vi "Dresden R2R Sputter 03.02.2018 IY24.vi"() -> ()   [LabVIEW 2009] (continued)
                                frame #0 {
                                n24699 = local write "Pc_bv1_auto_open"(TRUE ("Pc_bv1_auto_open")) -> ()
                                }
                                frame #1 {
                                }
                                }
                                }
                                frame #1 {
                                }
                                }
                                }
                                frame #4 {
                                n24700 = local read "Semi"() -> (w30074:bool)
                                n24701 = case shown="False" w30074 {
                                frame #0 {
                                n24702 = local read "Pc_bv_opened_ch1"() -> (w30075:bool)
                                n24703 = case shown="False" w30075 {
                                frame #0 {
                                n24704 = Wait (ms)(milliseconds to wait=u32 1000) -> ()  [unwired: 1 out]
                                }
                                frame #1 {
                                }
                                }
                                }
                                frame #1 {
                                }
                                }
                                }
                                frame #5 {
                                n24705 = local read "Semi"() -> (w30077:bool)
                                n24706 = case shown="False" w30077 {
                                frame #0 {
                                n24707 = while {
                                i -> [w30083]
                                stop <- w30079 stop-if-true
                                n24708 = local read "Pc_bv_opened_ch1"() -> (w30081:bool)
                                n24709 = Greater?(x=w30083, y=120) -> (0:w30082:bool)
                                n24710 = local read "Semi"() -> (w30080:bool)
                                n24711 = Compound Arithmetic op=OR(w30080, w30081, w30082) -> (w30079:bool)
                                n24712 = Wait (ms)(milliseconds to wait=u32 500) -> ()  [unwired: 1 out]
                                }
                                }
                                frame #1 {
                                }
                                }
                                }
                                frame #6 {
                                n24713 = local read "Semi"() -> (w30085:bool)
                                n24714 = case shown="False" w30085 {
                                frame #0 {
                                n24715 = local read "Pc_bv_opened_ch1"() -> (w30086:bool)
                                n24716 = case shown="False" w30086 {
                                frame #0 {
                                n24717 = local write "Error Message"("Start up process  cancelled\nbecause  PC-BV not opened.\nPlease check PC-BV1 connections." ("Error Message")) -> ()
                                n24718 = Wait (ms)(milliseconds to wait=u32 1000) -> ()  [unwired: 1 out]
                                }
                                frame #1 {
                                }
                                }
                                }
                                frame #1 {
                                }
                                }
                                }
                                }
                                }
                                frame #1 {
                                }
                                }
                                }
                                frame #1 {
                                n24719 = local read "Semi"() -> (w30089:bool)
                                n24720 = case shown="False" w30089 {
                                frame #0 {
                                n24721 = Wait (ms)(milliseconds to wait=u32 1000) -> ()  [unwired: 1 out]
                                n24722 = local write "SMW19"(TRUE ("CMW16")) -> ()
                                }
                                frame #1 {
                                }
                                }
                                }
                                }
                                }
                                frame #16 {
                                # "set ar zero"
                                n24723 = stacked-sequence {
                                frame #0 {
                                n24724 = local read "Semi"() -> (w30092:bool)
                                n24725 = case shown="False" w30092 {
                                frame #0 {
                                n24726 = stacked-sequence {
                                frame #0 {
                                n24727 = local read "Semi"() -> (w30093:bool)
                                n24728 = case shown="False" w30093 {
                                frame #0 {
                                n24729 = local write "Ar_auto_set_zero_ch1"(TRUE ("Ar_auto_set_zero_ch1")) -> ()
                                }
                                frame #1 {
                                }
                                }
                                }
                                frame #1 {
                                n24730 = local read "Semi"() -> (w30095:bool)
                                n24731 = case shown="False" w30095 {
                                frame #0 {
                                n24732 = while {
                                i -> [w30098]
                                stop <- w30097 stop-if-true
                                n24733 = Greater?(x=w30098, y=150) -> (0:w30097:bool)
                                n24734 = local read "Semi"() -> (w30096:bool)
                                n24735 = case shown="False" w30096 {
                                tunnel: [FALSE TRUE] -> _
                                frame #0 {
                                n24736 = Wait Until Next ms Multiple(millisecond multiple=u32 200) -> ()  [unwired: 1 out]
                                }
                                frame #1 {
                                }
                                }
                                }
                                }
                                frame #1 {
                                }
                                }
                                }
                                frame #2 {
                                n24737 = local read "Semi"() -> (w30103:bool)
                                n24738 = case shown="False" w30103 {
                                frame #0 {
                                n24739 = local read "Ar_sccm_act 5"() -> (w30105:dbl)
                                n24740 = Less?(x=w30105, y=1) -> (x < y?=w30104:bool)
                                n24741 = case shown="False" w30104 {
                                frame #0 {
                                n24742 = local write "Ar_auto_set_zero_ch1"(TRUE ("Ar_auto_set_zero_ch1")) -> ()
                                }
                                frame #1 {
                                }
                                }
                                }
                                frame #1 {
                                }
                                }
                                }
                                frame #3 {
                                n24743 = local read "Semi"() -> (w30108:bool)
                                n24744 = case shown="False" w30108 {
                                frame #0 {
                                n24745 = local read "Ar_sccm_act 5"() -> (w30110:dbl)
                                n24746 = Less?(x=w30110, y=1) -> (x < y?=w30109:bool)
                                n24747 = case shown="False" w30109 {
                                frame #0 {
                                n24748 = while {
                                i -> [w30116]
                                stop <- w30113 stop-if-true
                                n24749 = Greater?(x=w30116, y=150) -> (0:w30114:bool)
                                n24750 = local read "Semi"() -> (w30112:bool)
                                n24751 = case shown="True" w30112 {
                                tunnel: [FALSE FALSE] -> w30115
                                frame #0 {
                                }
                                frame #1 {
                                n24752 = Wait Until Next ms Multiple(millisecond multiple=u32 200) -> ()  [unwired: 1 out]
                                }
                                }
                                n24753 = Or(x=w30115, y=w30114) -> (x .or. y?=w30113:bool)
                                }
                                }
                                frame #1 {
                                }
                                }
                                }
                                frame #1 {
                                }
                                }
                                }
                                frame #4 {
                                n24754 = local read "Semi"() -> (w30121:bool)
                                n24755 = case shown="False" w30121 {
                                frame #0 {
                                n24756 = Wait (ms)(milliseconds to wait=u32 1000) -> ()  [unwired: 1 out]
                                n24757 = local write "SMW21"(TRUE ("CMW17")) -> ()
                                n24758 = local write "Ar_auto_set_zero_ch1"(FALSE ("Ar_auto_set_zero_ch1")) -> ()
                                }
                                frame #1 {
                                }
                                }
                                }
                                }
                                }
                                frame #1 {
                                }
                                }
                                }
                                frame #1 {
                                n24759 = local read "Semi"() -> (w30125:bool)
                                n24760 = case shown="False" w30125 {
                                frame #0 {
                                n24761 = Wait (ms)(milliseconds to wait=u32 1000) -> ()  [unwired: 1 out]
                                }
                                frame #1 {
                                }
                                }
                                }
                                }
                                }
                                frame #17 {
                                # "sov-ar close"
                                n24762 = stacked-sequence {
                                frame #0 {
                                n24763 = local read "Semi"() -> (w30127:bool)
                                n24764 = case shown="False" w30127 {
                                frame #0 {
                                n24765 = while {
                                i -> [w30133]
                                stop <- w30128 stop-if-true
                                n24766 = Greater?(x=w30133, y=50) -> (0:w30132:bool)
                                n24767 = case shown="True" w30132 {
                                frame #0 {
                                }
                                frame #1 {
                                n24768 = local write "Semi"(TRUE ("Semi")) -> ()
                                n24769 = local write "Error Message"("Coating Process  \nwas cancelled.\nPlease check \nSOV-Ar connection." ("Error Message")) -> ()
                                }
                                }
                                n24770 = local read "Ch1_Sov_Ar_di"() -> (w30131:bool)
                                n24771 = case shown="True" w30131 {
                                tunnel: [TRUE FALSE] -> w30130
                                frame #0 {
                                }
                                frame #1 {
                                n24772 = local write "Ch1_Sov_Ar_do"(FALSE ("Ch1_WFC_do")) -> ()
                                n24773 = Wait Until Next ms Multiple(millisecond multiple=u32 200) -> ()  [unwired: 1 out]
                                }
                                }
                                n24774 = local read "Semi"() -> (w30129:bool)
                                n24775 = Or(x=w30130, y=w30129) -> (x .or. y?=w30128:bool)
                                }
                                }
                                frame #1 {
                                }
                                }
                                }
                                frame #1 {
                                n24776 = local read "Semi"() -> (w30141:bool)
                                n24777 = case shown="False" w30141 {
                                frame #0 {
                                n24778 = local write "SMW22"(TRUE ("CMW2")) -> ()
                                n24779 = Wait (ms)(milliseconds to wait=u32 1000) -> ()  [unwired: 1 out]
                                }
                                frame #1 {
                                }
                                }
                                }
                                }
                                }
                                frame #18 {
                                # "ROLL FOR"
                                n24780 = stacked-sequence {
                                frame #0 {
                                n24781 = local read "R Single Microwave Number"() -> (w30146:dbl)
                                n24782 = Equal?(x=w30146, y=1.0) -> (x = y?=w30144:bool)
                                n24783 = case shown="True" w30144 {
                                frame #0 {
                                }
                                frame #1 {
                                n24784 = stacked-sequence {
                                frame #0 {
                                n24785 = local read "R Maximum diameter"() -> (w30151:dbl)
                                n24786 = local read "R Web speed(cm/min)"() -> (w30149:dbl)
                                n24787 = local read "R Minimum diameter"() -> (w30152:dbl)
                                n24788 = local read "R Web thicness"() -> (w30150:dbl)
                                n24789 = local read "R _Total_length"() -> (w30147:dbl)
                                n24790 = Wait (ms)(milliseconds to wait=u32 1000) -> ()  [unwired: 1 out]
                                n24791 = local write "Max Diameter"(w30151) -> ()
                                n24792 = local write "Web Thickness"(w30150) -> ()
                                n24793 = local write "Min Diameter"(w30152) -> ()
                                n24794 = local write "Web Speed"(w30149) -> ()
                                n24795 = local write "Region"(w30147) -> ()
                                }
                                frame #1 {
                                n24796 = local write "Calculate_auto"(TRUE ("Calculate_auto")) -> ()
                                n24797 = Wait (ms)(milliseconds to wait=u32 1000) -> ()  [unwired: 1 out]
                                }
                                frame #2 {
                                n24798 = local write "Roll_side_select"(enum32{"Left to Right", "Right to Left"}."Right to Left" ("Roll_side_select")) -> ()
                                }
                                frame #3 {
                                n24799 = local write "Parameters_auto_set"(TRUE ("Parameters_auto_set")) -> ()
                                }
                                frame #4 {
                                n24800 = while {
                                i -> [w30163]
                                stop <- w30158 stop-if-true
                                n24801 = Greater?(x=w30163, y=100) -> (0:w30159:bool)
                                n24802 = Wait Until Next ms Multiple(millisecond multiple=u32 300) -> ()  [unwired: 1 out]
                                n24803 = local read "Parameters_auto_set"() -> (w30157:bool)
                                n24804 = case shown="False" w30157 {
                                tunnel: [TRUE FALSE] -> w30160
                                frame #0 {
                                }
                                frame #1 {
                                }
                                }
                                n24805 = Or(x=w30160, y=w30159) -> (x .or. y?=w30158:bool)
                                }
                                }
                                frame #5 {
                                n24806 = local read "R Tension Value"() -> (w30167:dbl)
                                n24807 = Wait (ms)(milliseconds to wait=u32 1000) -> ()  [unwired: 1 out]
                                n24808 = local write "TC2_set_value"(w30167) -> ()
                                }
                                frame #6 {
                                n24809 = local write "TC2_auto_set"(TRUE ("TC1_auto_set")) -> ()
                                }
                                frame #7 {
                                w30169 = u16 0 items=["1", "2", "3", "4"] ("Target Chamber Sensor")
                                n24810 = local write "Target Chamber Sensor"(w30169) -> ()
                                }
                                frame #8 {
                                n24811 = local write "Start_roll"(TRUE ("Test_auto_start")) -> ()
                                n24812 = Wait (ms)(milliseconds to wait=u32 300) -> ()  [unwired: 1 out]
                                }
                                frame #9 {
                                n24813 = while {
                                stop <- w30173 stop-if-true
                                n24814 = local read "Actual Length"() -> (w30177:dbl)
                                n24815 = local read "Region"() -> (w30176:dbl)
                                n24816 = Greater Or Equal?(x=w30177, y=w30176) -> (x >= y?=w30174:bool)
                                n24817 = local read "Semi"() -> (w30175:bool)
                                n24818 = Or(x=w30174, y=w30175) -> (x .or. y?=w30173:bool)
                                n24819 = Wait Until Next ms Multiple(millisecond multiple=u32 300) -> ()  [unwired: 1 out]
                                }
                                }
                                frame #10 {
                                n24820 = local read "Semi"() -> (w30178:bool)
                                n24821 = case shown="False" w30178 {
                                frame #0 {
                                n24822 = Wait (ms)(milliseconds to wait=u32 1000) -> ()  [unwired: 1 out]
                                n24823 = local write "SMW15"(TRUE ("CMW12")) -> ()
                                }
                                frame #1 {
                                }
                                }
                                }
                                }
                                }
                                }
                                }
                                frame #1 {
                                n24824 = local read "Semi"() -> (w30181:bool)
                                n24825 = case shown="False" w30181 {
                                frame #0 {
                                n24826 = Wait (ms)(milliseconds to wait=u32 1000) -> ()  [unwired: 1 out]
                                n24827 = local write "SMW23"(TRUE ("CMW19")) -> ()
                                }
                                frame #1 {
                                }
                                }
                                }
                                }
                                }
                                frame #19 {
                                # "CC CLOSE"
                                n24828 = stacked-sequence {
                                frame #0 {
                                n24829 = local read "Semi"() -> (w30184:bool)
                                n24830 = case shown="False" w30184 {
                                frame #0 {
                                n24831 = while {
                                i -> [w30190]
                                stop <- w30185 stop-if-true
                                n24832 = Greater?(x=w30190, y=50) -> (0:w30189:bool)
                                n24833 = case shown="True" w30189 {
                                frame #0 {
                                }
                                frame #1 {
                                n24834 = local write "Semi"(TRUE ("Semi")) -> ()
                                n24835 = local write "Error Message"("Coating Process  \nwas cancelled.\nPlease check \nBG-BV connection." ("Error Message")) -> ()
                                }
                                }
                                n24836 = local read "Ch1_Cc_on_off_di"() -> (w30188:bool)
                                n24837 = case shown="False" w30188 {
                                tunnel: [FALSE TRUE] -> w30187
                                frame #0 {
                                n24838 = local write "Ch1_Cc_on_off_do"(TRUE ("Ch1_WFC_do")) -> ()
                                n24839 = Wait Until Next ms Multiple(millisecond multiple=u32 200) -> ()  [unwired: 1 out]
                                }
                                frame #1 {
                                }
                                }
                                n24840 = local read "Semi"() -> (w30186:bool)
                                n24841 = Or(x=w30187, y=w30186) -> (x .or. y?=w30185:bool)
                                }
                                }
                                frame #1 {
                                }
                                }
                                }
                                frame #1 {
                                n24842 = local read "Semi"() -> (w30198:bool)
                                n24843 = case shown="False" w30198 {
                                frame #0 {
                                n24844 = local write "SMW24"(TRUE ("SMW24")) -> ()
                                n24845 = Wait (ms)(milliseconds to wait=u32 1000) -> ()  [unwired: 1 out]
                                }
                                frame #1 {
                                }
                                }
                                }
                                }
                                }
                                frame #20 {
                                # "BG-BV close"
                                n24846 = stacked-sequence {
                                frame #0 {
                                n24847 = local read "Semi"() -> (w30201:bool)
                                n24848 = case shown="False" w30201 {
                                frame #0 {
                                n24849 = while {
                                i -> [w30207]
                                stop <- w30202 stop-if-true
                                n24850 = Greater?(x=w30207, y=50) -> (0:w30206:bool)
                                n24851 = case shown="True" w30206 {
                                frame #0 {
                                }
                                frame #1 {
                                n24852 = local write "Semi"(TRUE ("Semi")) -> ()
                                n24853 = local write "Error Message"("Coating Process  \nwas cancelled.\nPlease check \nBG-BV connection." ("Error Message")) -> ()
                                }
                                }
                                n24854 = local read "Ch1_Bg_bv_di"() -> (w30205:bool)
                                n24855 = case shown="False" w30205 {
                                tunnel: [FALSE TRUE] -> w30204
                                frame #0 {
                                n24856 = local write "Ch1_Bg_bv_do"(TRUE ("Ch1_WFC_do")) -> ()
                                n24857 = Wait Until Next ms Multiple(millisecond multiple=u32 200) -> ()  [unwired: 1 out]
                                }
                                frame #1 {
                                }
                                }
                                n24858 = local read "Semi"() -> (w30203:bool)
                                n24859 = Or(x=w30204, y=w30203) -> (x .or. y?=w30202:bool)
                                }
                                }
                                frame #1 {
                                }
                                }
                                }
                                frame #1 {
                                n24860 = local read "Semi"() -> (w30215:bool)
                                n24861 = case shown="False" w30215 {
                                frame #0 {
                                n24862 = local write "SMW25"(TRUE ("CMW2")) -> ()
                                n24863 = Wait (ms)(milliseconds to wait=u32 1000) -> ()  [unwired: 1 out]
                                }
                                frame #1 {
                                }
                                }
                                }
                                }
                                }
                                frame #21 {
                                n24864 = local read "Semi"() -> (w30218:bool)
                                n24865 = case shown="False" w30218 {
                                frame #0 {
                                n24866 = local write "Cnt_Do_Buzzer"(TRUE ("CMW20")) -> ()
                                n24867 = local write "SMW26"(TRUE ("CMW20")) -> ()
                                n24868 = Wait (ms)(milliseconds to wait=u32 2500) -> ()  [unwired: 1 out]
                                }
                                frame #1 {
                                }
                                }
                                }
                                frame #22 {
                                n24869 = local read "Semi"() -> (w30222:bool)
                                n24870 = case shown="False" w30222 {
                                frame #0 {
                                n24871 = local write "Cnt_Do_Buzzer"(FALSE ("CMW20")) -> ()
                                n24872 = Wait (ms)(milliseconds to wait=u32 1000) -> ()  [unwired: 1 out]
                                }
                                frame #1 {
                                }
                                }
                                }
                                }
                                }
                                frame #1 {
                                }
                              }
                            }
                          }
                        }
                        frame #1 {
                          n24873 = local read "R_DC_Chamber_selection"() -> (w30225:enum32{"Chamber II", "Chamber III"})
                          n24874 = case shown="\"Chamber III\"" w30225 {
                            frame #0 {
                              n24875 = local read "Single_Ch2_Interlock"() -> (w30226:dbl)
                              n24876 = local read "Ch2_pressure"() -> (w30230:dbl)
                              n24877 = local read "started_up_ch2"() -> (w30228:bool)
                              n24878 = In Range and Coerce(upper limit=w30226, x=w30230, lower limit=1e-08) -> (In Range?=w30231:bool)  [unwired: 1 out]
                              n24879 = And(x=w30231, y=w30228) -> (x .and. y?=w30227:bool)
                              n24880 = case shown="True" w30227 {
                                frame #0 {
                                }
                                frame #1 {
                                n24881 = local read "Semi"() -> (w30232:bool)
                                n24882 = case shown="False" w30232 {
                                frame #0 {
                                n24883 = stacked-sequence {
                                frame #0 {
                                n24884 = stacked-sequence {
                                frame #0 {
                                n24885 = local read "Semi"() -> (w30233:bool)
                                n24886 = case shown="False" w30233 {
                                frame #0 {
                                w30236 = FALSE ("Casette_servo_start/stop_do")
                                n24887 = local write "Ch2_Sov_Ar_do"(FALSE ("Ch1_Sov_Ar_do")) -> ()
                                n24888 = local write "Dc_host_auto"(TRUE ("Dc_host_auto")) -> ()
                                n24889 = local write "Ar_auto_set_zero_ch2"(TRUE ("Dc_auto_set_zero")) -> ()
                                n24890 = local write "final_process_messages"("Coating was Completed" ("final_process_messages")) -> ()
                                n24891 = local write "system_status"("Coating Mode is Active" ("system_status")) -> ()
                                n24892 = local write "Casette_servo_start/stop_do"(w30236) -> ()
                                n24893 = local write "Tension_controllers_start/stop_do"(w30236) -> ()
                                }
                                frame #1 {
                                }
                                }
                                }
                                frame #1 {
                                n24894 = local read "Semi"() -> (w30240:bool)
                                n24895 = case shown="False" w30240 {
                                frame #0 {
                                n24896 = Wait (ms)(milliseconds to wait=u32 2500) -> ()  [unwired: 1 out]
                                }
                                frame #1 {
                                }
                                }
                                }
                                frame #2 {
                                n24897 = local read "Semi"() -> (w30242:bool)
                                n24898 = case shown="False" w30242 {
                                frame #0 {
                                n24899 = local write "Ch2_SRV_start_stop_do"(FALSE ("Ch1_SRV_start_stop_do")) -> ()
                                }
                                frame #1 {
                                }
                                }
                                }
                                frame #3 {
                                n24900 = local read "Semi"() -> (w30244:bool)
                                n24901 = case shown="False" w30244 {
                                frame #0 {
                                n24902 = Wait (ms)(milliseconds to wait=u32 2500) -> ()  [unwired: 1 out]
                                }
                                frame #1 {
                                }
                                }
                                }
                                frame #4 {
                                n24903 = local read "Semi"() -> (w30246:bool)
                                n24904 = case shown="False" w30246 {
                                frame #0 {
                                n24905 = Wait (ms)(milliseconds to wait=u32 1000) -> ()  [unwired: 1 out]
                                n24906 = local write "SDC1 1"(TRUE ("CMW1")) -> ()
                                }
                                frame #1 {
                                }
                                }
                                }
                                }
                                }
                                frame #1 {
                                n24907 = local read "ch_present_position"() -> (w30251:dbl)
                                n24908 = Not Equal?(x=w30251, y=2.0) -> (x != y?=w30249:bool)
                                n24909 = case shown="True" w30249 {
                                frame #0 {
                                }
                                frame #1 {
                                n24910 = stacked-sequence {
                                frame #0 {
                                n24911 = local write "Set chamber"(2.0 ("Set chamber")) -> ()
                                n24912 = Wait (ms)(milliseconds to wait=u32 100) -> ()  [unwired: 1 out]
                                }
                                frame #1 {
                                n24913 = local write "Auto_set_transfer"(TRUE ("Auto_set_transfer")) -> ()
                                }
                                frame #2 {
                                n24914 = while {
                                stop <- w30256 stop-if-true
                                n24915 = Wait Until Next ms Multiple(millisecond multiple=u32 300) -> ()  [unwired: 1 out]
                                n24916 = local read "Auto_set_transfer"() -> (w30257:bool)
                                n24917 = local read "Semi"() -> (w30259:bool)
                                n24918 = Not(x=w30257) -> (.not. x?=w30258:bool)
                                n24919 = Or(x=w30258, y=w30259) -> (x .or. y?=w30256:bool)
                                }
                                }
                                frame #3 {
                                n24920 = local write "SDC1 12"(TRUE ("SMW1 2")) -> ()
                                n24921 = Wait (ms)(milliseconds to wait=u32 300) -> ()  [unwired: 1 out]
                                }
                                }
                                }
                                }
                                }
                                frame #2 {
                                # "WATER FLOW CONTROL OPEN"
                                n24922 = stacked-sequence {
                                frame #0 {
                                n24923 = local read "Semi"() -> (w30262:bool)
                                n24924 = case shown="False" w30262 {
                                frame #0 {
                                n24925 = while {
                                i -> [w30268]
                                stop <- w30263 stop-if-true
                                n24926 = Greater?(x=w30268, y=100) -> (0:w30267:bool)
                                n24927 = case shown="True" w30267 {
                                frame #0 {
                                }
                                frame #1 {
                                n24928 = local write "Semi"(TRUE ("Semi")) -> ()
                                n24929 = local write "Error Message"("Coating Process  \nwas cancelled.\nPlease check water \nflow connection." ("Error Message")) -> ()
                                }
                                }
                                n24930 = local read "Ch4_WFS_di"() -> (w30266:bool)
                                n24931 = case shown="True" w30266 {
                                tunnel: [TRUE FALSE] -> w30265
                                frame #0 {
                                }
                                frame #1 {
                                n24932 = local write "Ch4_WFC_do"(FALSE ("Ch1_WFC_do")) -> ()
                                n24933 = Wait Until Next ms Multiple(millisecond multiple=u32 200) -> ()  [unwired: 1 out]
                                }
                                }
                                n24934 = local read "Semi"() -> (w30264:bool)
                                n24935 = Or(x=w30265, y=w30264) -> (x .or. y?=w30263:bool)
                                }
                                }
                                frame #1 {
                                }
                                }
                                }
                                frame #1 {
                                n24936 = local read "Semi"() -> (w30276:bool)
                                n24937 = case shown="False" w30276 {
                                frame #0 {
                                n24938 = while {
                                i -> [w30282]
                                stop <- w30277 stop-if-true
                                n24939 = Greater?(x=w30282, y=100) -> (0:w30281:bool)
                                n24940 = case shown="True" w30281 {
                                frame #0 {
                                }
                                frame #1 {
                                n24941 = local write "Semi"(TRUE ("Semi")) -> ()
                                n24942 = local write "Error Message"("Coating Process  \nwas cancelled.\nPlease check water \nflow connection." ("Error Message")) -> ()
                                }
                                }
                                n24943 = local read "Ch3_WFS_di"() -> (w30280:bool)
                                n24944 = case shown="True" w30280 {
                                tunnel: [TRUE FALSE] -> w30279
                                frame #0 {
                                }
                                frame #1 {
                                n24945 = local write "Ch3_WFC_do"(FALSE ("Ch1_WFC_do")) -> ()
                                n24946 = Wait Until Next ms Multiple(millisecond multiple=u32 200) -> ()  [unwired: 1 out]
                                }
                                }
                                n24947 = local read "Semi"() -> (w30278:bool)
                                n24948 = Or(x=w30279, y=w30278) -> (x .or. y?=w30277:bool)
                                }
                                }
                                frame #1 {
                                }
                                }
                                }
                                frame #2 {
                                n24949 = local read "Semi"() -> (w30290:bool)
                                n24950 = case shown="False" w30290 {
                                frame #0 {
                                n24951 = while {
                                i -> [w30296]
                                stop <- w30291 stop-if-true
                                n24952 = Greater?(x=w30296, y=100) -> (0:w30295:bool)
                                n24953 = case shown="True" w30295 {
                                frame #0 {
                                }
                                frame #1 {
                                n24954 = local write "Semi"(TRUE ("Semi")) -> ()
                                n24955 = local write "Error Message"("Coating Process  \nwas cancelled.\nPlease check water \nflow connection." ("Error Message")) -> ()
                                }
                                }
                                n24956 = local read "Ch1_WFS_di"() -> (w30294:bool)
                                n24957 = case shown="True" w30294 {
                                tunnel: [TRUE FALSE] -> w30293
                                frame #0 {
                                }
                                frame #1 {
                                n24958 = local write "Ch1_WFC_do"(FALSE ("Ch1_WFC_do")) -> ()
                                n24959 = Wait Until Next ms Multiple(millisecond multiple=u32 200) -> ()  [unwired: 1 out]
                                }
                                }
                                n24960 = local read "Semi"() -> (w30292:bool)
                                n24961 = Or(x=w30293, y=w30292) -> (x .or. y?=w30291:bool)
                                }
                                }
                                frame #1 {
                                }
                                }
                                }
                                frame #3 {
                                n24962 = local read "Semi"() -> (w30304:bool)
                                n24963 = case shown="False" w30304 {
                                frame #0 {
                                n24964 = while {
                                i -> [w30310]
                                stop <- w30305 stop-if-true
                                n24965 = Greater?(x=w30310, y=100) -> (0:w30309:bool)
                                n24966 = case shown="True" w30309 {
                                frame #0 {
                                }
                                frame #1 {
                                n24967 = local write "Semi"(TRUE ("Semi")) -> ()
                                n24968 = local write "Error Message"("Coating Process  \nwas cancelled.\nPlease check water \nflow connection." ("Error Message")) -> ()
                                }
                                }
                                n24969 = local read "Ch2_WFS_di"() -> (w30308:bool)
                                n24970 = case shown="False" w30308 {
                                tunnel: [FALSE TRUE] -> w30307
                                frame #0 {
                                n24971 = local write "Ch2_WFC_do"(TRUE ("Ch1_WFC_do")) -> ()
                                n24972 = Wait Until Next ms Multiple(millisecond multiple=u32 200) -> ()  [unwired: 1 out]
                                }
                                frame #1 {
                                }
                                }
                                n24973 = local read "Semi"() -> (w30306:bool)
                                n24974 = Or(x=w30307, y=w30306) -> (x .or. y?=w30305:bool)
                                }
                                }
                                frame #1 {
                                }
                                }
                                }
                                frame #4 {
                                n24975 = local read "Semi"() -> (w30318:bool)
                                n24976 = case shown="False" w30318 {
                                frame #0 {
                                n24977 = local write "SDC1 2"(TRUE ("SDC1 2")) -> ()
                                n24978 = Wait (ms)(milliseconds to wait=u32 1000) -> ()  [unwired: 1 out]
                                }
                                frame #1 {
                                }
                                }
                                }
                                }
                                }
                                frame #3 {
                                # "BG-BV open"
                                n24979 = stacked-sequence {
                                frame #0 {
                                n24980 = local read "Semi"() -> (w30321:bool)
                                n24981 = case shown="False" w30321 {
                                frame #0 {
                                n24982 = while {
                                i -> [w30327]
                                stop <- w30322 stop-if-true
                                n24983 = Greater?(x=w30327, y=50) -> (0:w30326:bool)
                                n24984 = case shown="True" w30326 {
                                frame #0 {
                                }
                                frame #1 {
                                n24985 = local write "Semi"(TRUE ("Semi")) -> ()
                                n24986 = local write "Error Message"("Coating Process  \nwas cancelled.\nPlease check \nBG-BV connection." ("Error Message")) -> ()
                                }
                                }
                                n24987 = local read "Ch2_Bg_bv_di"() -> (w30325:bool)
                                n24988 = case shown="False" w30325 {
                                tunnel: [FALSE TRUE] -> w30324
                                frame #0 {
                                n24989 = local write "Ch2_Bg_bv_do"(TRUE ("Ch1_WFC_do")) -> ()
                                n24990 = Wait Until Next ms Multiple(millisecond multiple=u32 200) -> ()  [unwired: 1 out]
                                }
                                frame #1 {
                                }
                                }
                                n24991 = local read "Semi"() -> (w30323:bool)
                                n24992 = Or(x=w30324, y=w30323) -> (x .or. y?=w30322:bool)
                                }
                                }
                                frame #1 {
                                }
                                }
                                }
                                frame #1 {
                                n24993 = local read "Semi"() -> (w30335:bool)